vi "Velociprobe_Nanopositioner_Control_RT.vi"() -> ()   [LabVIEW 2015] (continued)
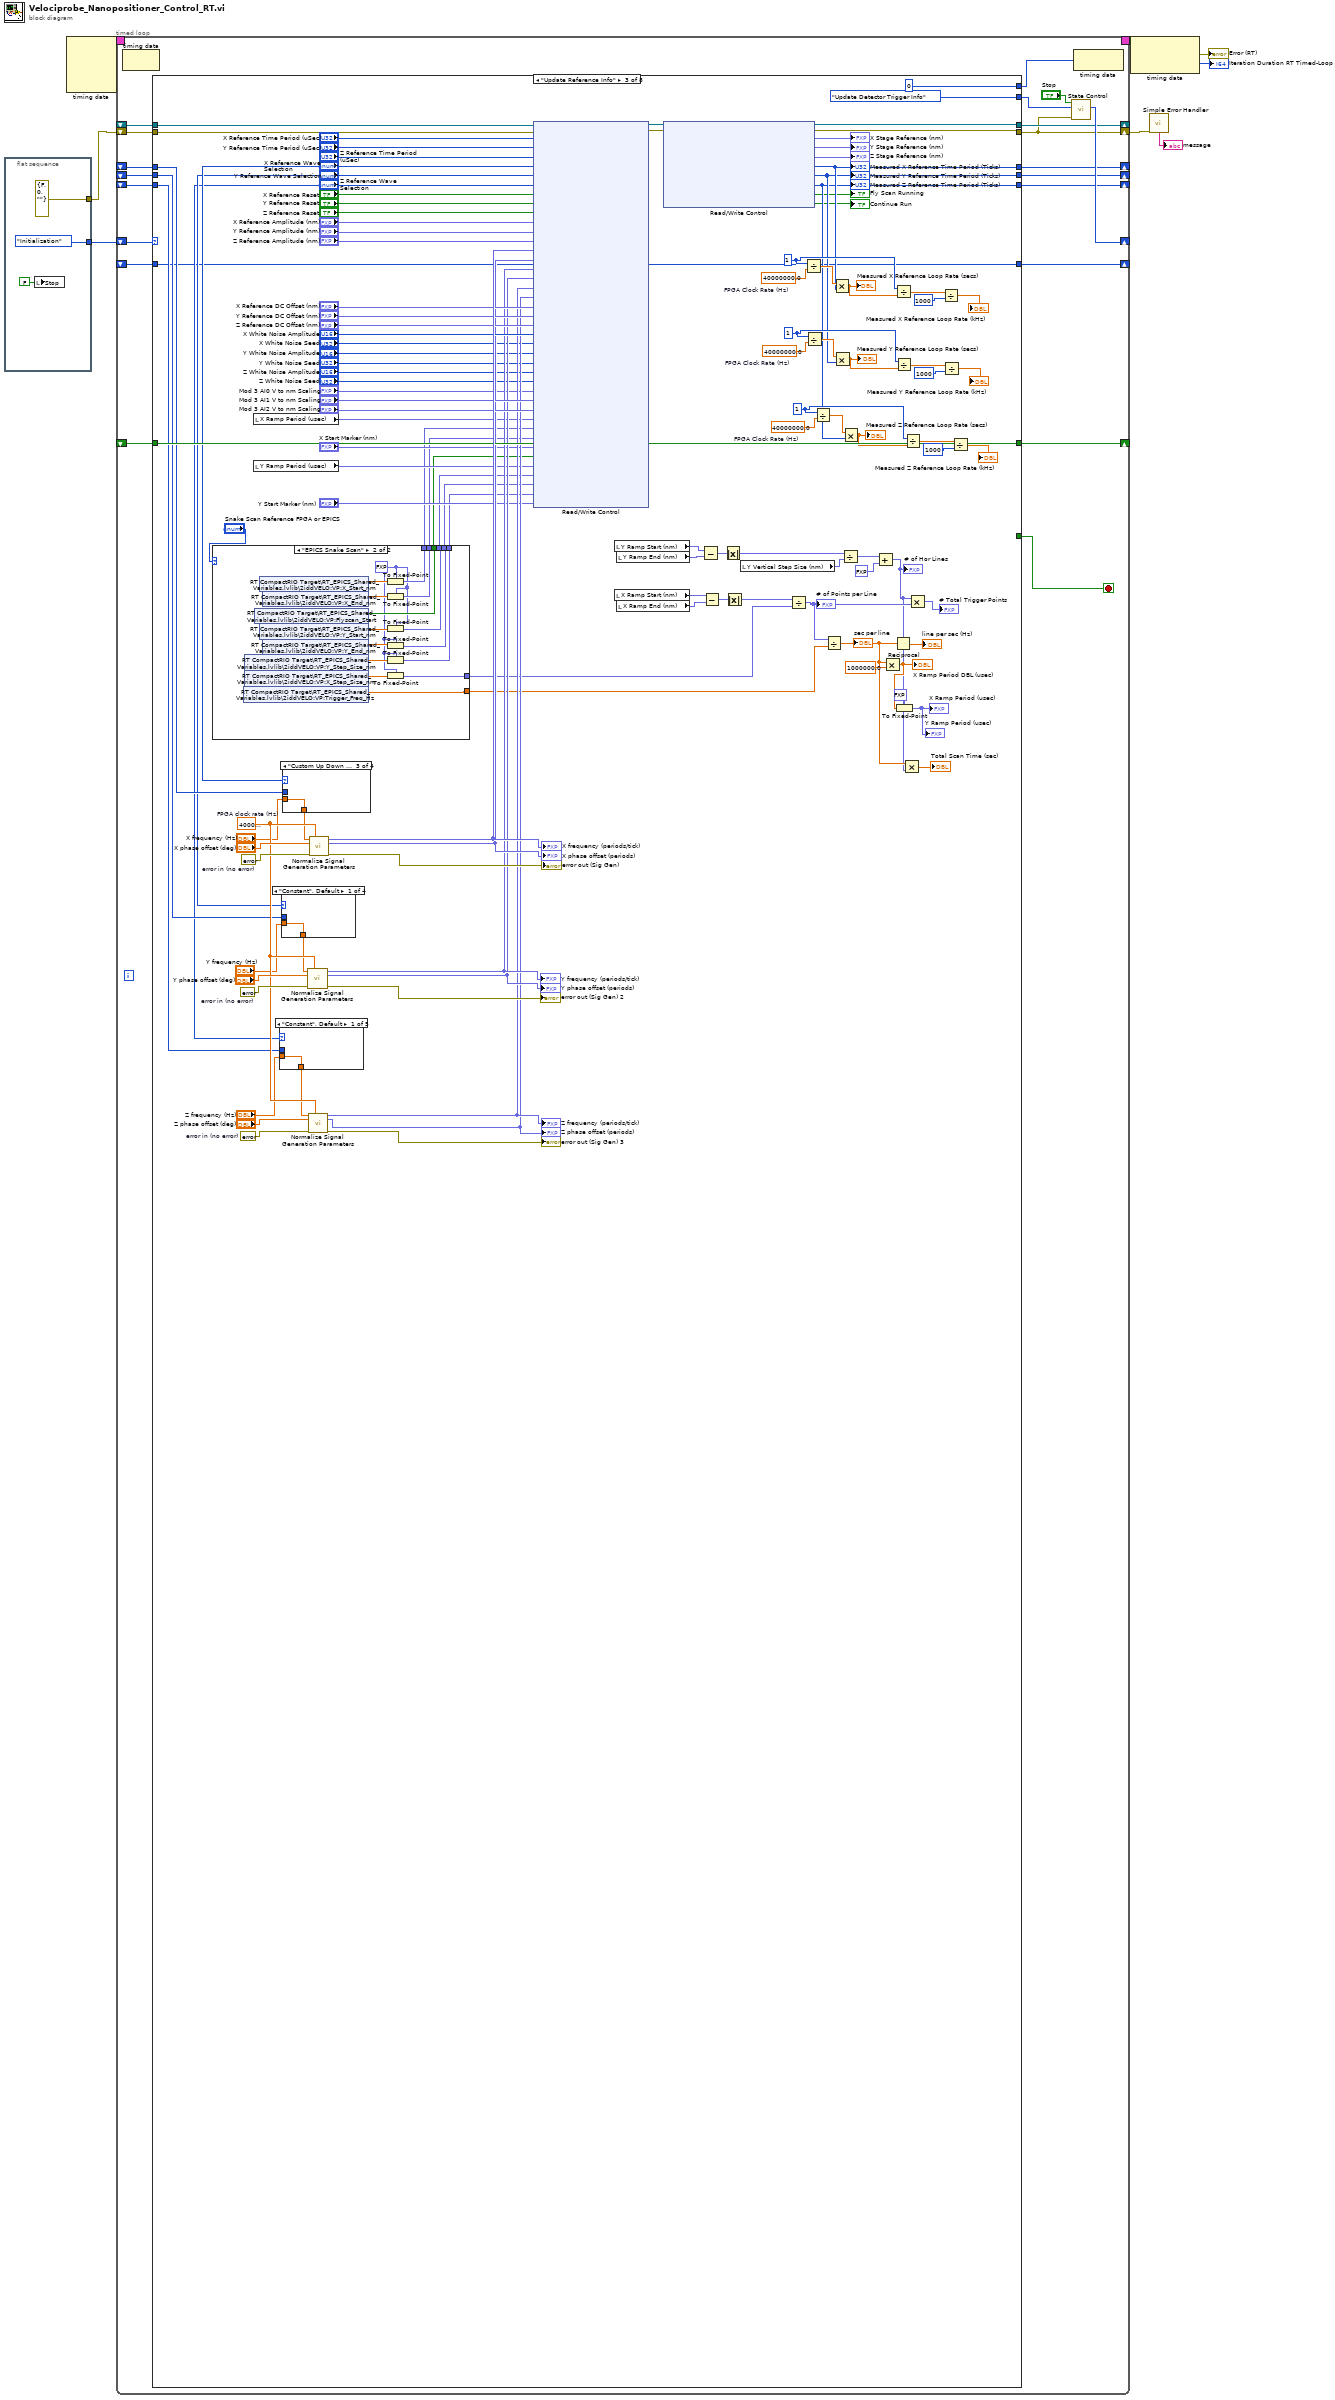
[diagram p0: block diagram]
diagram:
  n1 = flat-sequence {
    tunnel: [State_Enum."Initialization" ("States")] -> w6
    tunnel: [errorcluster {"status"=FALSE, "code"=0, "source"=""} ("error constant")] -> w2
    frame #0 {
      n2 = local write "Stop"(FALSE ("Stop")) -> ()
    }
  }
  n3 = node-c288() -> (w8:T8)  [unwired: 4 in]
  n4 = timed-loop {
    timing: w8 -> [_]
    timing-out: [_] -> w7
    shift-right: [w30] -> _
    shift-left: _ -> [w29]
    shift-right: [w24] -> _
    shift-left: w6 -> [w28]
    shift-right: [w23] -> _
    shift-left: _ -> [w22]
    shift-right: [w21] -> _
    shift-left: _ -> [w20]
    shift-right: [w18] -> _
    shift-left: _ -> [w19]
    shift-right: [w17] -> _
    shift-left: _ -> [w16]
    shift-right: [w15] -> _
    shift-left: _ -> [w12]
    shift-right: [w14] -> w1
    shift-left: w2 -> [w13]
    stop <- w27 stop-if-true
    n5 = node-c288() -> ()  [unwired: 1 in, 1 out]
    n6 = case shown="\"Update Reference Info\"" w28 {
      tunnel: [i64 0 i64 0 i64 0 i64 0 i64 0 i64 0 i64 0 i64 0] -> w31
      tunnel: [w51 w345 w628 w727 w768 w802 "Write Data" w895] -> w30
      tunnel: w29 -> [w51 w345 w628 w727 w768 w802 w848 w895]
      tunnel: [State_Enum."Update Controller Info" State_Enum."Update Reference Info" State_Enum."Update Detector Trigger Info" State_Enum."Update Datalog Info" ("States") State_Enum."Check FPGA Status" State_Enum."Reading FIFO" State_Enum."Update Controller Info" State_Enum."Initialization"] -> w25
      tunnel: [_ _ _ _ _ _ _ w896] -> w27
      tunnel: [w49 w74 w584 w722 w749 w801 w839 w894] -> w23
      tunnel: w22 -> [w49 w74 w583 w722 w749 w801 w839 w894]
      tunnel: [w48 w73 w580 w721 w748 w800 w838 w893] -> w21
      tunnel: w20 -> [w48 w73 w578 w721 w748 w800 w838 w893]
      tunnel: w19 -> [w47 w72 w575 w720 w747 w799 w837 w892]
      tunnel: [w47 w72 w579 w720 w747 w799 w837 w892] -> w18
      tunnel: [w46 w71 w570 w703 w746 w798 w822 w891] -> w17
      tunnel: w16 -> [w46 w71 w570 w702 w746 w798 w822 w891]
      tunnel: [w35 w66 w530 w694 w740 w795 w816 w886] -> w15
      tunnel: [w33 w65 w531 w693 w741 w793 w814 w884] -> w14
      tunnel: w13 -> [w32 w70 w534 w697 w744 w796 w819 w889]
      tunnel: w12 -> [_ w69 w535 w698 w745 w797 w820 w890]
      frame "Initialization", Default {
        w54 = 0  # IRQ Number(s)
        n7 = xnode "Open FPGA VI Reference"("error in"=w32, "resource name"=tag "rio://169.254.76.54/RIO0") -> ("FPGA VI Reference Out"=w44:refnum<k20>, "error out"=w45:errorcluster)
        n8 = xnode "Invoke Method"("FPGA VI Reference In"=w44, "error in"=w45, "Requested Depth"="Requested Depth") -> ("FPGA VI Reference Out"=w43:refnum<k20>, "error out"=w42:errorcluster, "Actual Depth"=→"Actual Depth":u32)
        n9 = xnode "Read/Write Control"("FPGA VI Reference In"=w43, "error in"=w42, "Datalog Time Period (uSec)"="Datalog Time Period (uSec)", "Datalog Cases"="Datalog Cases", "Interrupt Boolean"=FALSE) -> ("FPGA VI Reference Out"=w41:refnum<k20>, "error out"=w40:errorcluster)
        n10 = xnode "Invoke Method"("FPGA VI Reference In"=w41, "error in"=w40, "IRQ Number(s)"=w54, "Timeout (ms)"="IRQ Timeout (ms)") -> ("FPGA VI Reference Out"=w39:refnum<k20>, "error out"=w38:errorcluster, "Timed Out"=→"IRQ Timed Out":bool, "IRQ(s) Asserted"=w56:i32)
        n11 = xnode "Invoke Method"("FPGA VI Reference In"=w39, "error in"=w38, "IRQ Number(s)"=w56) -> ("FPGA VI Reference Out"=w37:refnum<k20>, "error out"=w36:errorcluster)
        n12 = xnode "Read/Write Control"("FPGA VI Reference In"=w37, "error in"=w36) -> ("FPGA VI Reference Out"=w35:refnum<k20>, "error out"=w34:errorcluster, "error out (FPGA)"=w57:errorcluster)
        n13 = invoke on="Waveform Graph 2" class="WFGraph (strict)" method="Reinit To Default"() -> (error out=w50:errorcluster)  [unwired: 3 in, 2 out]
        n14 = Merge Errors "Merge Errors"(w34, w57, w50) -> (w33:errorcluster)
      }
      frame "Update Controller Info" {
        w294 = dbl[] [1.0, 2.0, 4.0, 5.0]  # Index_soscoeff_zz1
        w133 = dbl[] [1.0, 2.0, 4.0, 5.0]  # Index_soscoeff_yz1
        w154 = dbl[] [1.0, 2.0, 4.0, 5.0]  # Index_soscoeff_xz1
        w185 = dbl[] [1.0, 2.0, 4.0, 5.0]  # Index_soscoeff_zy1
        w315 = dbl[] [1.0, 2.0, 4.0, 5.0]  # Index_soscoeff_yy1
        w206 = dbl[] [1.0, 2.0, 4.0, 5.0]  # Index_soscoeff_xy1
        w232 = dbl[] [1.0, 2.0, 4.0, 5.0]  # Index_soscoeff_zx1
        w341 = dbl[] [1.0, 2.0, 4.0, 5.0]  # Index_soscoeff_xx1
        w258 = dbl[] [1.0, 2.0, 4.0, 5.0]  # Index_soscoeff_yx1
        w114 = "%.10f"  # format (%.3f)
        w122 = "%.10f"  # format (%.3f)
        w135 = "%.10f"  # format (%.3f)
        w143 = "%.10f"  # format (%.3f)
        w166 = "%.10f"  # format (%.3f)
        w174 = "%.10f"  # format (%.3f)
        w187 = "%.10f"  # format (%.3f)
        w195 = "%.10f"  # format (%.3f)
        w213 = "%.10f"  # format (%.3f)
        w221 = "%.10f"  # format (%.3f)
        w239 = "%.10f"  # format (%.3f)
        w247 = "%.10f"  # format (%.3f)
        w275 = "%.10f"  # format (%.3f)
        w283 = "%.10f"  # format (%.3f)
        w296 = "%.10f"  # format (%.3f)
        w304 = "%.10f"  # format (%.3f)
        w105 = fxp<+/-,42,9> 0.0 ("fixed-point type")
        w317 = "%.10f"  # format (%.3f)
        w104 = fxp<+/-,64,9> 0.0 ("fixed-point type")
        w330 = "%.10f"  # format (%.3f)
        w349 = 40000000.0  # FPGA Clock Rate (Hz)
        w81 = 1
        n15 = local read "sos gain SF Controller yy1c"() -> (w269:fxp<+/-,42,9>)
        n16 = local read "sos gain SF Controller yz1c"() -> (w90:fxp<+/-,42,9>)
        n17 = local read "sos gain SF Controller yx1c"() -> (w236:fxp<+/-,42,9>)
        n18 = local read "sos gain SF Controller xy1c"() -> (w159:fxp<+/-,42,9>)
        n19 = local read "sos gain SF Controller zy1c"() -> (w164:fxp<+/-,42,9>)
        n20 = local read "sos gain SF Controller xz1c"() -> (w106:fxp<+/-,42,9>)
        n21 = local read "sos gain SF Controller xx1c"() -> (w319:fxp<+/-,42,9>)
        n22 = local read "sos gain SF Controller zz1c"() -> (w267:fxp<+/-,42,9>)
        n23 = local read "sos gain SF Controller zx1c"() -> (w211:fxp<+/-,42,9>)
        n24 = local read "-a01(2) yy1c"() -> (w273:fxp<+/-,64,9>[])
        n25 = local read "-a02(2) yy1c"() -> (w272:fxp<+/-,64,9>[])
        n26 = local read "-a01(2) yz1c"() -> (w111:fxp<+/-,64,9>[])
        n27 = local read "-a02(2) yz1c"() -> (w112:fxp<+/-,64,9>[])
        n28 = local read "-a01(2) yx1c"() -> (w237:fxp<+/-,64,9>[])
        n29 = local read "-a02(2) yx1c"() -> (w233:fxp<+/-,64,9>[])
        n30 = local read "-a01(2) xy1c"() -> (w155:fxp<+/-,64,9>[])
        n31 = local read "-a02(2) xy1c"() -> (w156:fxp<+/-,64,9>[])
        n32 = local read "-a01(2) zy1c"() -> (w160:fxp<+/-,64,9>[])
        n33 = local read "-a02(2) zy1c"() -> (w161:fxp<+/-,64,9>[])
        n34 = local read "-a01(2) xz1c"() -> (w110:fxp<+/-,64,9>[])
        n35 = local read "-a02(2) xz1c"() -> (w109:fxp<+/-,64,9>[])
        n36 = local read "-a01(2) xx1c"() -> (w328:fxp<+/-,64,9>[])
        n37 = local read "-a02(2) xx1c"() -> (w327:fxp<+/-,64,9>[])
        n38 = local read "-a01(2) zz1c"() -> (w268:fxp<+/-,64,9>[])
        n39 = local read "-a02(2) zz1c"() -> (w264:fxp<+/-,64,9>[])
        n40 = local read "-a01(2) zx1c"() -> (w207:fxp<+/-,64,9>[])
        n41 = local read "-a02(2) zx1c"() -> (w208:fxp<+/-,64,9>[])
        n42 = local read "b01(2) yy1c"() -> (w271:fxp<+/-,64,9>[])
        n43 = local read "b02(2) yy1c"() -> (w270:fxp<+/-,64,9>[])
        n44 = local read "b01(2) yz1c"() -> (w76:fxp<+/-,64,9>[])
        n45 = local read "b02(2) yz1c"() -> (w75:fxp<+/-,64,9>[])
        n46 = local read "b01(2) yx1c"() -> (w234:fxp<+/-,64,9>[])
        n47 = local read "b02(2) yx1c"() -> (w235:fxp<+/-,64,9>[])
        n48 = local read "b01(2) xy1c"() -> (w157:fxp<+/-,64,9>[])
        n49 = local read "b02(2) xy1c"() -> (w158:fxp<+/-,64,9>[])
        n50 = local read "b01(2) zy1c"() -> (w162:fxp<+/-,64,9>[])
        n51 = local read "b02(2) zy1c"() -> (w163:fxp<+/-,64,9>[])
        n52 = local read "b01(2) xz1c"() -> (w108:fxp<+/-,64,9>[])
        n53 = local read "b02(2) xz1c"() -> (w107:fxp<+/-,64,9>[])
        n54 = local read "b01(2) xx1c"() -> (w326:fxp<+/-,64,9>[])
        n55 = local read "b02(2) xx1c"() -> (w325:fxp<+/-,64,9>[])
        n56 = local read "b01(2) zz1c"() -> (w265:fxp<+/-,64,9>[])
        n57 = local read "b02(2) zz1c"() -> (w266:fxp<+/-,64,9>[])
        n58 = local read "b01(2) zx1c"() -> (w209:fxp<+/-,64,9>[])
        n59 = local read "b02(2) zx1c"() -> (w210:fxp<+/-,64,9>[])
        n60 = Or(x="Optics Z Reset", y="Reset All") -> (x .or. y?=w103:bool)
        n61 = Or(x="Sample Z Reset", y="Reset All") -> (x .or. y?=w100:bool)
        n62 = Or(x="Optics X Reset", y="Reset All") -> (x .or. y?=w262:bool)
        n63 = Or(x="Optics Y Reset", y="Reset All") -> (x .or. y?=w260:bool)
        n64 = Or(x="Sample X Reset", y="Reset All") -> (x .or. y?=w102:bool)
        n65 = Or(x="Sample Y Reset", y="Reset All") -> (x .or. y?=w101:bool)
        n66 = call-poly <vilib>:"Read Delimited Spreadsheet.vi"("file path (dialog if empty)"="file path soscoeff_xx1", "format (%.3f)"=w330) -> ("all rows"=w329:dbl[][])  [unwired: 8 in, 5 out]
        n67 = call-poly <vilib>:"Read Delimited Spreadsheet.vi"("file path (dialog if empty)"="file path soscoeff_zy1", "format (%.3f)"=w174) -> ("all rows"=w173:dbl[][])  [unwired: 8 in, 5 out]
        n68 = call-poly <vilib>:"Read Delimited Spreadsheet.vi"("file path (dialog if empty)"="file path soscoeff_xy1", "format (%.3f)"=w195) -> ("all rows"=w194:dbl[][])  [unwired: 8 in, 5 out]
        n69 = call-poly <vilib>:"Read Delimited Spreadsheet.vi"("file path (dialog if empty)"="file path soscoeff_zx1", "format (%.3f)"=w221) -> ("all rows"=w220:dbl[][])  [unwired: 8 in, 5 out]
        n70 = call-poly <vilib>:"Read Delimited Spreadsheet.vi"("file path (dialog if empty)"="file path soscoeff_xz1", "format (%.3f)"=w143) -> ("all rows"=w142:dbl[][])  [unwired: 8 in, 5 out]
        n71 = call-poly <vilib>:"Read Delimited Spreadsheet.vi"("file path (dialog if empty)"="file path soscoeff_yx1", "format (%.3f)"=w247) -> ("all rows"=w246:dbl[][])  [unwired: 8 in, 5 out]
        n72 = call-poly <vilib>:"Read Delimited Spreadsheet.vi"("file path (dialog if empty)"="file path soscoeff_yy1", "format (%.3f)"=w304) -> ("all rows"=w303:dbl[][])  [unwired: 8 in, 5 out]
        n73 = call-poly <vilib>:"Read Delimited Spreadsheet.vi"("file path (dialog if empty)"="file path soscoeff_yz1", "format (%.3f)"=w122) -> ("all rows"=w121:dbl[][])  [unwired: 8 in, 5 out]
        n74 = call-poly <vilib>:"Read Delimited Spreadsheet.vi"("file path (dialog if empty)"="file path soscoeff_zz1", "format (%.3f)"=w283) -> ("all rows"=w282:dbl[][])  [unwired: 8 in, 5 out]
        n75 = Transpose 2D Array(2D array=w329) -> (transposed array=w340:dbl[][])
        n76 = Transpose 2D Array(2D array=w173) -> (transposed array=w184:dbl[][])
        n77 = Transpose 2D Array(2D array=w194) -> (transposed array=w205:dbl[][])
        n78 = Transpose 2D Array(2D array=w220) -> (transposed array=w231:dbl[][])
        n79 = Transpose 2D Array(2D array=w142) -> (transposed array=w153:dbl[][])
        n80 = Transpose 2D Array(2D array=w246) -> (transposed array=w257:dbl[][])
        n81 = Transpose 2D Array(2D array=w303) -> (transposed array=w314:dbl[][])
        n82 = Transpose 2D Array(2D array=w121) -> (transposed array=w132:dbl[][])
        n83 = Transpose 2D Array(2D array=w282) -> (transposed array=w293:dbl[][])
        n84 = call-poly <vilib>:"Read Delimited Spreadsheet.vi"("file path (dialog if empty)"="file path sos gain SF Controller_xx1", "format (%.3f)"=w317) -> ("all rows"=w316:dbl[][])  [unwired: 8 in, 5 out]
        n85 = call-poly <vilib>:"Read Delimited Spreadsheet.vi"("file path (dialog if empty)"="file path sos gain SF Controller_zy1", "format (%.3f)"=w166) -> ("all rows"=w165:dbl[][])  [unwired: 8 in, 5 out]
        n86 = call-poly <vilib>:"Read Delimited Spreadsheet.vi"("file path (dialog if empty)"="file path sos gain SF Controller_xy1", "format (%.3f)"=w187) -> ("all rows"=w186:dbl[][])  [unwired: 8 in, 5 out]
        n87 = call-poly <vilib>:"Read Delimited Spreadsheet.vi"("file path (dialog if empty)"="file path sos gain SF Controller_zx1", "format (%.3f)"=w213) -> ("all rows"=w212:dbl[][])  [unwired: 8 in, 5 out]
        n88 = call-poly <vilib>:"Read Delimited Spreadsheet.vi"("file path (dialog if empty)"="file path sos gain SF Controller_xz1", "format (%.3f)"=w135) -> ("all rows"=w134:dbl[][])  [unwired: 8 in, 5 out]
        n89 = call-poly <vilib>:"Read Delimited Spreadsheet.vi"("file path (dialog if empty)"="file path sos gain SF Controller_yx1", "format (%.3f)"=w239) -> ("all rows"=w238:dbl[][])  [unwired: 8 in, 5 out]
        n90 = call-poly <vilib>:"Read Delimited Spreadsheet.vi"("file path (dialog if empty)"="file path sos gain SF Controller_yy1", "format (%.3f)"=w296) -> ("all rows"=w295:dbl[][])  [unwired: 8 in, 5 out]
        n91 = call-poly <vilib>:"Read Delimited Spreadsheet.vi"("file path (dialog if empty)"="file path sos gain SF Controller_yz1", "format (%.3f)"=w114) -> ("all rows"=w113:dbl[][])  [unwired: 8 in, 5 out]
        n92 = call-poly <vilib>:"Read Delimited Spreadsheet.vi"("file path (dialog if empty)"="file path sos gain SF Controller_zz1", "format (%.3f)"=w275) -> ("all rows"=w274:dbl[][])  [unwired: 8 in, 5 out]
        n93 = xnode "Read/Write Control"("FPGA VI Reference In"=w69, "error in"=w70, "Controller Time Period (uSec)"="Controller Time Period (uSec)", "Controller Output Time Period (uSec)"="Controller Output Time Period (uSec)", "System Loop Type"="System Loop Type", "Controller Output Upper Limit"="Controller Output Upper Limit", "Controller Output Lower Limit"="Controller Output Lower Limit", "X-Stage nm to V Scaling"="X-Stage nm to V Scaling", "X-Stage Scaling Direction"="X-Stage Scaling Direction", "Y-Stage nm to V Scaling"="Y-Stage nm to V Scaling", "Z-Stage nm to V Scaling"="Z-Stage nm to V Scaling", "Plant Output Time Period (uSec)"="Plant Output Time Period (uSec)", "Reset Optics X"=w262, "Reset Optics Y"=w260, "Reset Optics Z"=w103, "Reset Sample X"=w102, "Reset Sample Y"=w101, "Reset Sample Z"=w100, "Optics X Stage Resolution (nm)"="Optics X Stage Resolution (nm)", "Optics Y Stage Resolution (nm)"="Optics Y Stage Resolution (nm)", "Optics Z Stage Resolution (nm)"="Optics Z Stage Resolution (nm)", "Sample X Stage Resolution (nm)"="Sample X Stage Resolution (nm)", "Sample Y Stage Resolution (nm)"="Sample Y Stage Resolution (nm)", "Sample Z Stage Resolution (nm)"="Sample Z Stage Resolution (nm)", "Scaling mV to V"="Scaling mV to V", "-a01(2) xx1"=w328, "-a02(2) xx1"=w327, "b01(2) xx1"=w326, "b02(2) xx1"=w325, "sos gain SF Controller xx1"=w319, "-a01(2) yy1"=w273, "-a02(2) yy1"=w272, "b01(2) yy1"=w271, "b02(2) yy1"=w270, "sos gain SF Controller yy1"=w269, "-a01(2) zz1"=w268, "-a02(2) zz1"=w264, "b01(2) zz1"=w265, "b02(2) zz1"=w266, "sos gain SF Controller zz1"=w267, "-a01(2) yx1"=w237, "-a02(2) yx1"=w233, "b01(2) yx1"=w234, "b02(2) yx1"=w235, "sos gain SF Controller yx1"=w236, "-a01(2) zx1"=w207, "-a02(2) zx1"=w208, "b01(2) zx1"=w209, "b02(2) zx1"=w210, "sos gain SF Controller zx1"=w211, "-a01(2) xy1"=w155, "-a02(2) xy1"=w156, "b01(2) xy1"=w157, "b02(2) xy1"=w158, "sos gain SF Controller xy1"=w159, "-a01(2) zy1"=w160, "-a02(2) zy1"=w161, "b01(2) zy1"=w162, "b02(2) zy1"=w163, "sos gain SF Controller zy1"=w164, "-a01(2) xz1"=w110, "-a02(2) xz1"=w109, "b01(2) xz1"=w108, "b02(2) xz1"=w107, "sos gain SF Controller xz1"=w106, "-a01(2) yz1"=w111, "-a02(2) yz1"=w112, "b01(2) yz1"=w76, "b02(2) yz1"=w75, "sos gain SF Controller yz1"=w90, "Analog Input Time Period (uSec)"="Analog Input Time Period (uSec)", "Optics and or Sample Stage"="Optics and or Sample Stage", "Y-Stage Scaling Direction"="Y-Stage Scaling Direction", "Z-Stage Scaling Direction"="Z-Stage Scaling Direction") -> ("FPGA VI Reference Out"=w68:refnum<k20>, "error out"=w67:errorcluster)
        n94 = for {
          tunnel: w341 -> [w518] mode=indexing
          tunnel: w340 -> [w517]
          tunnel: [w516] -> _ mode=indexing
          shift-right: [w516] -> w332
          shift-left: _ -> [w515]
          shift-left: _ -> [w514]
          shift-left: _ -> [w513]
          tunnel: [w515] -> w333
          tunnel: [w514] -> w334
          tunnel: [w513] -> w335
          n95 = Index Array "Index Array"(array=w517, index (row)=w518) -> (element=w516:dbl[])  [unwired: 1 in]
        }
        n96 = Index Array(array=w316, index (row)=0 ("index (row) 6")) -> (element=w324:dbl[])  [unwired: 1 in]
        n97 = for {
          tunnel: w185 -> [w416] mode=indexing
          tunnel: w184 -> [w415]
          tunnel: [w414] -> _ mode=indexing
          shift-right: [w414] -> w176
          shift-left: _ -> [w413]
          shift-left: _ -> [w412]
          shift-left: _ -> [w411]
          tunnel: [w413] -> w177
          tunnel: [w412] -> w178
          tunnel: [w411] -> w179
          n98 = Index Array "Index Array"(array=w415, index (row)=w416) -> (element=w414:dbl[])  [unwired: 1 in]
        }
        n99 = Index Array(array=w165, index (row)=0 ("index (row) 18")) -> (element=w172:dbl[])  [unwired: 1 in]
        n100 = for {
          tunnel: w206 -> [w433] mode=indexing
          tunnel: w205 -> [w432]
          tunnel: [w431] -> _ mode=indexing
          shift-right: [w431] -> w197
          shift-left: _ -> [w430]
          shift-left: _ -> [w429]
          shift-left: _ -> [w428]
          tunnel: [w430] -> w198
          tunnel: [w429] -> w199
          tunnel: [w428] -> w200
          n101 = Index Array "Index Array"(array=w432, index (row)=w433) -> (element=w431:dbl[])  [unwired: 1 in]
        }
        n102 = Index Array(array=w186, index (row)=0 ("index (row) 16")) -> (element=w193:dbl[])  [unwired: 1 in]
        n103 = for {
          tunnel: w232 -> [w450] mode=indexing
          tunnel: w231 -> [w449]
          tunnel: [w448] -> _ mode=indexing
          shift-right: [w448] -> w223
          shift-left: _ -> [w447]
          shift-left: _ -> [w446]
          shift-left: _ -> [w445]
          tunnel: [w447] -> w224
          tunnel: [w446] -> w225
          tunnel: [w445] -> w226
          n104 = Index Array "Index Array"(array=w449, index (row)=w450) -> (element=w448:dbl[])  [unwired: 1 in]
        }
        n105 = Index Array(array=w212, index (row)=0 ("index (row) 14")) -> (element=w219:dbl[])  [unwired: 1 in]
        n106 = for {
          tunnel: w154 -> [w399] mode=indexing
          tunnel: w153 -> [w398]
          tunnel: [w397] -> _ mode=indexing
          shift-right: [w397] -> w145
          shift-left: _ -> [w396]
          shift-left: _ -> [w395]
          shift-left: _ -> [w394]
          tunnel: [w396] -> w146
          tunnel: [w395] -> w147
          tunnel: [w394] -> w148
          n107 = Index Array "Index Array"(array=w398, index (row)=w399) -> (element=w397:dbl[])  [unwired: 1 in]
        }
        n108 = Index Array(array=w134, index (row)=0 ("index (row) 20")) -> (element=w141:dbl[])  [unwired: 1 in]
        n109 = for {
          tunnel: w258 -> [w467] mode=indexing
          tunnel: w257 -> [w466]
          tunnel: [w465] -> _ mode=indexing
          shift-right: [w465] -> w249
          shift-left: _ -> [w464]
          shift-left: _ -> [w463]
          shift-left: _ -> [w462]
          tunnel: [w464] -> w250
          tunnel: [w463] -> w251
          tunnel: [w462] -> w252
          n110 = Index Array "Index Array"(array=w466, index (row)=w467) -> (element=w465:dbl[])  [unwired: 1 in]
        }
        n111 = Index Array(array=w238, index (row)=0 ("index (row) 12")) -> (element=w245:dbl[])  [unwired: 1 in]
        n112 = for {
          tunnel: w315 -> [w501] mode=indexing
          tunnel: w314 -> [w500]
          tunnel: [w499] -> _ mode=indexing
          shift-right: [w499] -> w306
          shift-left: _ -> [w498]
          shift-left: _ -> [w497]
          shift-left: _ -> [w496]
          tunnel: [w498] -> w307
          tunnel: [w497] -> w308
          tunnel: [w496] -> w309
          n113 = Index Array "Index Array"(array=w500, index (row)=w501) -> (element=w499:dbl[])  [unwired: 1 in]
        }
        n114 = Index Array(array=w295, index (row)=0 ("index (row) 8")) -> (element=w302:dbl[])  [unwired: 1 in]
        n115 = for {
          tunnel: w133 -> [w382] mode=indexing
          tunnel: w132 -> [w381]
          tunnel: [w380] -> _ mode=indexing
          shift-right: [w380] -> w124
          shift-left: _ -> [w379]
          shift-left: _ -> [w378]
          shift-left: _ -> [w377]
          tunnel: [w379] -> w125
          tunnel: [w378] -> w126
          tunnel: [w377] -> w127
          n116 = Index Array "Index Array"(array=w381, index (row)=w382) -> (element=w380:dbl[])  [unwired: 1 in]
        }
        n117 = Index Array(array=w113, index (row)=0 ("index (row) 22")) -> (element=w120:dbl[])  [unwired: 1 in]
        n118 = Index Array(array=w274, index (row)=0 ("index (row) 10")) -> (element=w281:dbl[])  [unwired: 1 in]
        n119 = for {
          tunnel: w294 -> [w484] mode=indexing
          tunnel: w293 -> [w483]
          tunnel: [w482] -> _ mode=indexing
          shift-right: [w482] -> w285
          shift-left: _ -> [w481]
          shift-left: _ -> [w480]
          shift-left: _ -> [w479]
          tunnel: [w481] -> w286
          tunnel: [w480] -> w287
          tunnel: [w479] -> w288
          n120 = Index Array "Index Array"(array=w483, index (row)=w484) -> (element=w482:dbl[])  [unwired: 1 in]
        }
        n121 = Index Array(array=w324, index=0 ("index (row) 7")) -> (element=w322:dbl)
        n122 = Index Array(array=w172, index=0 ("index (row) 19")) -> (element=w170:dbl)
        n123 = Index Array(array=w193, index=0 ("index (row) 17")) -> (element=w191:dbl)
        n124 = Index Array(array=w219, index=0 ("index (row) 15")) -> (element=w217:dbl)
        n125 = Index Array(array=w141, index=0 ("index (row) 21")) -> (element=w139:dbl)
        n126 = Index Array(array=w245, index=0 ("index (row) 13")) -> (element=w243:dbl)
        n127 = Index Array(array=w302, index=0 ("index (row) 9")) -> (element=w300:dbl)
        n128 = Index Array(array=w120, index=0 ("index (row) 23")) -> (element=w118:dbl)
        n129 = Index Array(array=w281, index=0 ("index (row) 11")) -> (element=w279:dbl)
        n130 = xnode "Read/Write Control"("FPGA VI Reference In"=w68, "error in"=w67) -> ("FPGA VI Reference Out"=w66:refnum<k20>, "error out"=w65:errorcluster, "PI X-Stage Input (V)"=→"PI X-Stage Input (V)":fxp<+/-,20,5>, "PI Y-Stage Input (V)"=→"PI Y-Stage Input (V)":fxp<+/-,20,5>, "PI Z-Stage Input (V)"=→"PI Z-Stage Input (V)":fxp<+/-,20,5>, "X-Stage Input In Range?"=→"X-Stage Input In Range?":bool, "Y-Stage Input In Range?"=→"Y-Stage Input In Range?":bool, "Z-Stage Input In Range?"=→"Z-Stage Input In Range?":bool, "Measured Controller Time Period (Ticks)"=w350:u32, "Measured Controller Output Time Period (Ticks)"=w347:u32, "Measured Plant Output Time Period (Ticks)"=w82:u32, "Measured Analog Input Time Period (Ticks)"=→"Measured Analog Input Time Period (Ticks)":u32)
        "Measured Controller Time Period (Ticks)" <- w350
        "Measured Controller Output Time Period (Ticks)" <- w347
        "Measured Plant Output Time Period (Ticks)" <- w82
        n131 = To Fixed-Point(fixed-point type=w105, number=w191) -> (fixed-point=→"sos gain SF Controller xy1c":fxp<+/-,42,9>)
        n132 = To Fixed-Point(fixed-point type=w105, number=w300) -> (fixed-point=→"sos gain SF Controller yy1c":fxp<+/-,42,9>)
        n133 = To Fixed-Point(fixed-point type=w105, number=w170) -> (fixed-point=→"sos gain SF Controller zy1c":fxp<+/-,42,9>)
        n134 = To Fixed-Point(fixed-point type=w105, number=w139) -> (fixed-point=→"sos gain SF Controller xz1c":fxp<+/-,42,9>)
        n135 = To Fixed-Point(fixed-point type=w105, number=w118) -> (fixed-point=→"sos gain SF Controller yz1c":fxp<+/-,42,9>)
        n136 = To Fixed-Point(fixed-point type=w105, number=w243) -> (fixed-point=→"sos gain SF Controller yx1c":fxp<+/-,42,9>)
        n137 = To Fixed-Point(fixed-point type=w105, number=w217) -> (fixed-point=→"sos gain SF Controller zx1c":fxp<+/-,42,9>)
        n138 = To Fixed-Point(fixed-point type=w105, number=w279) -> (fixed-point=→"sos gain SF Controller zz1c":fxp<+/-,42,9>)
        n139 = To Fixed-Point(fixed-point type=w105, number=w322) -> (fixed-point=→"sos gain SF Controller xx1c":fxp<+/-,42,9>)
        n140 = Divide(x=w81, y=w349) -> (x/y=w83:dbl)
        n141 = Multiply(x=w83, y=w350) -> (x*y=w351:dbl)
        "Measured Controller Loop Rate (secs)" <- w351
        n142 = Multiply(x=w83, y=w347) -> (x*y=w359:dbl)
        "Measured Controller Output Loop Rate (secs)" <- w359
        n143 = Multiply(x=w83, y=w82) -> (x*y=w355:dbl)
        "Measured Plant Output Loop Rate (secs)" <- w355
        n144 = Multiply(x=w83, y=w82) -> (x*y=w87:dbl)
        "Measured Analog Input Loop Rate (secs)" <- w87
        n145 = for {
          tunnel: w177 -> [w427] mode=indexing
          tunnel: [w426] -> w183 mode=indexing
          tunnel: w176 -> [w425] mode=indexing
          tunnel: w179 -> [w424] mode=indexing
          tunnel: w178 -> [w423] mode=indexing
          tunnel: [w422] -> w182 mode=indexing
          tunnel: [w421] -> w181 mode=indexing
          tunnel: [w420] -> w180 mode=indexing
          tunnel: w104 -> [w417]
          n146 = Negate(x=w427) -> (-x=w419:dbl)
          n147 = Negate(x=w425) -> (-x=w418:dbl)
          n148 = To Fixed-Point(fixed-point type=w417, number=w419) -> (fixed-point=w426:fxp<+/-,64,9>)
          n149 = To Fixed-Point(fixed-point type=w417, number=w418) -> (fixed-point=w422:fxp<+/-,64,9>)
          n150 = To Fixed-Point(fixed-point type=w417, number=w424) -> (fixed-point=w421:fxp<+/-,64,9>)
          n151 = To Fixed-Point(fixed-point type=w417, number=w423) -> (fixed-point=w420:fxp<+/-,64,9>)
        }
        "-a01(2) zy1c" <- w183
        "-a02(2) zy1c" <- w182
        "b01(2) zy1c" <- w181
        "b02(2) zy1c" <- w180
        n152 = for {
          tunnel: w333 -> [w529] mode=indexing
          tunnel: [w528] -> w339 mode=indexing
          tunnel: w332 -> [w527] mode=indexing
          tunnel: w335 -> [w526] mode=indexing
          tunnel: w334 -> [w525] mode=indexing
          tunnel: [w524] -> w338 mode=indexing
          tunnel: [w523] -> w337 mode=indexing
          tunnel: [w522] -> w336 mode=indexing
          tunnel: w104 -> [w519]
          n153 = Negate(x=w529) -> (-x=w521:dbl)
          n154 = Negate(x=w527) -> (-x=w520:dbl)
          n155 = To Fixed-Point(fixed-point type=w519, number=w521) -> (fixed-point=w528:fxp<+/-,64,9>)
          n156 = To Fixed-Point(fixed-point type=w519, number=w520) -> (fixed-point=w524:fxp<+/-,64,9>)
          n157 = To Fixed-Point(fixed-point type=w519, number=w526) -> (fixed-point=w523:fxp<+/-,64,9>)
          n158 = To Fixed-Point(fixed-point type=w519, number=w525) -> (fixed-point=w522:fxp<+/-,64,9>)
        }
        "-a01(2) xx1c" <- w339
        "-a02(2) xx1c" <- w338
        "b01(2) xx1c" <- w337
        "b02(2) xx1c" <- w336
        n159 = for {
          tunnel: w198 -> [w444] mode=indexing
          tunnel: [w443] -> w204 mode=indexing
          tunnel: w197 -> [w442] mode=indexing
          tunnel: w200 -> [w441] mode=indexing
          tunnel: w199 -> [w440] mode=indexing
          tunnel: [w439] -> w203 mode=indexing
          tunnel: [w438] -> w202 mode=indexing
          tunnel: [w437] -> w201 mode=indexing
          tunnel: w104 -> [w434]
          n160 = Negate(x=w444) -> (-x=w436:dbl)
          n161 = Negate(x=w442) -> (-x=w435:dbl)
          n162 = To Fixed-Point(fixed-point type=w434, number=w436) -> (fixed-point=w443:fxp<+/-,64,9>)
          n163 = To Fixed-Point(fixed-point type=w434, number=w435) -> (fixed-point=w439:fxp<+/-,64,9>)
          n164 = To Fixed-Point(fixed-point type=w434, number=w441) -> (fixed-point=w438:fxp<+/-,64,9>)
          n165 = To Fixed-Point(fixed-point type=w434, number=w440) -> (fixed-point=w437:fxp<+/-,64,9>)
        }
        "-a01(2) xy1c" <- w204
        "-a02(2) xy1c" <- w203
        "b01(2) xy1c" <- w202
        "b02(2) xy1c" <- w201
        n166 = for {
          tunnel: w146 -> [w410] mode=indexing
          tunnel: [w409] -> w152 mode=indexing
          tunnel: w145 -> [w408] mode=indexing
          tunnel: w148 -> [w407] mode=indexing
          tunnel: w147 -> [w406] mode=indexing
          tunnel: [w405] -> w151 mode=indexing
          tunnel: [w404] -> w150 mode=indexing
          tunnel: [w403] -> w149 mode=indexing
          tunnel: w104 -> [w400]
          n167 = Negate(x=w410) -> (-x=w402:dbl)
          n168 = Negate(x=w408) -> (-x=w401:dbl)
          n169 = To Fixed-Point(fixed-point type=w400, number=w402) -> (fixed-point=w409:fxp<+/-,64,9>)
          n170 = To Fixed-Point(fixed-point type=w400, number=w401) -> (fixed-point=w405:fxp<+/-,64,9>)
          n171 = To Fixed-Point(fixed-point type=w400, number=w407) -> (fixed-point=w404:fxp<+/-,64,9>)
          n172 = To Fixed-Point(fixed-point type=w400, number=w406) -> (fixed-point=w403:fxp<+/-,64,9>)
        }
        "-a01(2) xz1c" <- w152
        "-a02(2) xz1c" <- w151
        "b01(2) xz1c" <- w150
        "b02(2) xz1c" <- w149
        n173 = for {
          tunnel: w307 -> [w512] mode=indexing
          tunnel: [w511] -> w313 mode=indexing
          tunnel: w306 -> [w510] mode=indexing
          tunnel: w309 -> [w509] mode=indexing
          tunnel: w308 -> [w508] mode=indexing
          tunnel: [w507] -> w312 mode=indexing
          tunnel: [w506] -> w311 mode=indexing
          tunnel: [w505] -> w310 mode=indexing
          tunnel: w104 -> [w502]
          n174 = Negate(x=w512) -> (-x=w504:dbl)
          n175 = Negate(x=w510) -> (-x=w503:dbl)
          n176 = To Fixed-Point(fixed-point type=w502, number=w504) -> (fixed-point=w511:fxp<+/-,64,9>)
          n177 = To Fixed-Point(fixed-point type=w502, number=w503) -> (fixed-point=w507:fxp<+/-,64,9>)
          n178 = To Fixed-Point(fixed-point type=w502, number=w509) -> (fixed-point=w506:fxp<+/-,64,9>)
          n179 = To Fixed-Point(fixed-point type=w502, number=w508) -> (fixed-point=w505:fxp<+/-,64,9>)
        }
        "-a01(2) yy1c" <- w313
        "-a02(2) yy1c" <- w312
        "b01(2) yy1c" <- w311
        "b02(2) yy1c" <- w310
        n180 = for {
          tunnel: w224 -> [w461] mode=indexing
          tunnel: [w460] -> w230 mode=indexing
          tunnel: w223 -> [w459] mode=indexing
          tunnel: w226 -> [w458] mode=indexing
          tunnel: w225 -> [w457] mode=indexing
          tunnel: [w456] -> w229 mode=indexing
          tunnel: [w455] -> w228 mode=indexing
          tunnel: [w454] -> w227 mode=indexing
          tunnel: w104 -> [w451]
          n181 = Negate(x=w461) -> (-x=w453:dbl)
          n182 = Negate(x=w459) -> (-x=w452:dbl)
          n183 = To Fixed-Point(fixed-point type=w451, number=w453) -> (fixed-point=w460:fxp<+/-,64,9>)
          n184 = To Fixed-Point(fixed-point type=w451, number=w452) -> (fixed-point=w456:fxp<+/-,64,9>)
          n185 = To Fixed-Point(fixed-point type=w451, number=w458) -> (fixed-point=w455:fxp<+/-,64,9>)
          n186 = To Fixed-Point(fixed-point type=w451, number=w457) -> (fixed-point=w454:fxp<+/-,64,9>)
        }
        "-a01(2) zx1c" <- w230
        "-a02(2) zx1c" <- w229
        "b01(2) zx1c" <- w228
        "b02(2) zx1c" <- w227
        n187 = for {
          tunnel: w250 -> [w478] mode=indexing
          tunnel: [w477] -> w256 mode=indexing
          tunnel: w249 -> [w476] mode=indexing
          tunnel: w252 -> [w475] mode=indexing
          tunnel: w251 -> [w474] mode=indexing
          tunnel: [w473] -> w255 mode=indexing
          tunnel: [w472] -> w254 mode=indexing
          tunnel: [w471] -> w253 mode=indexing
          tunnel: w104 -> [w468]
          n188 = Negate(x=w478) -> (-x=w470:dbl)
          n189 = Negate(x=w476) -> (-x=w469:dbl)
          n190 = To Fixed-Point(fixed-point type=w468, number=w470) -> (fixed-point=w477:fxp<+/-,64,9>)
          n191 = To Fixed-Point(fixed-point type=w468, number=w469) -> (fixed-point=w473:fxp<+/-,64,9>)
          n192 = To Fixed-Point(fixed-point type=w468, number=w475) -> (fixed-point=w472:fxp<+/-,64,9>)
          n193 = To Fixed-Point(fixed-point type=w468, number=w474) -> (fixed-point=w471:fxp<+/-,64,9>)
        }
        "-a01(2) yx1c" <- w256
        "-a02(2) yx1c" <- w255
        "b01(2) yx1c" <- w254
        "b02(2) yx1c" <- w253
        n194 = for {
          tunnel: w125 -> [w393] mode=indexing
          tunnel: [w392] -> w131 mode=indexing
          tunnel: w124 -> [w391] mode=indexing
          tunnel: w127 -> [w390] mode=indexing
          tunnel: w126 -> [w389] mode=indexing
          tunnel: [w388] -> w130 mode=indexing
          tunnel: [w387] -> w129 mode=indexing
          tunnel: [w386] -> w128 mode=indexing
          tunnel: w104 -> [w383]
          n195 = Negate(x=w393) -> (-x=w385:dbl)
          n196 = Negate(x=w391) -> (-x=w384:dbl)
          n197 = To Fixed-Point(fixed-point type=w383, number=w385) -> (fixed-point=w392:fxp<+/-,64,9>)
          n198 = To Fixed-Point(fixed-point type=w383, number=w384) -> (fixed-point=w388:fxp<+/-,64,9>)
          n199 = To Fixed-Point(fixed-point type=w383, number=w390) -> (fixed-point=w387:fxp<+/-,64,9>)
          n200 = To Fixed-Point(fixed-point type=w383, number=w389) -> (fixed-point=w386:fxp<+/-,64,9>)
        }
        "-a01(2) yz1c" <- w131
        "-a02(2) yz1c" <- w130
        "b01(2) yz1c" <- w129
        "b02(2) yz1c" <- w128
        n201 = Divide(x=w81, y=w351) -> (x/y=w362:dbl)
        n202 = Divide(x=w81, y=w359) -> (x/y=w358:dbl)
        n203 = Divide(x=w81, y=w355) -> (x/y=w354:dbl)
        n204 = for {
          tunnel: w286 -> [w495] mode=indexing
          tunnel: [w494] -> w292 mode=indexing
          tunnel: w285 -> [w493] mode=indexing
          tunnel: w288 -> [w492] mode=indexing